vi "TLB Native Dynamic Events ver 0.26e.vi"() -> ()   [LabVIEW 2018] (continued)
          tunnel: w309 -> [_ _ _ _ _ _ _ _ _ _ _ _ _ _ _ _ _ _ _ _ _ _ _ _ _ _ _ _ _ _ _ _ _ _ _ _ _ _ _ _ _ _ _ _ _ _ _ _ _ _ _ _ _ _ _ _ _ _ _]
          tunnel: w308 -> [_ _ _ _ _ _ _ _ _ _ _ _ _ _ _ _ _ _ _ _ _ _ _ _ _ _ _ _ _ _ _ _ _ _ _ _ _ _ _ _ _ _ _ _ _ _ _ _ _ _ _ _ _ _ _ _ _ _ _]
          tunnel: w307 -> [_ _ _ _ _ _ _ _ _ _ _ _ _ _ _ _ _ _ _ _ _ _ _ _ _ _ _ _ _ _ _ _ _ _ _ _ _ _ _ _ _ _ _ _ _ _ _ _ _ _ _ _ _ _ _ _ _ _ _]
          tunnel: w306 -> [_ _ _ _ _ _ _ _ _ _ _ _ _ _ _ _ _ _ _ _ _ _ _ _ _ _ _ _ _ _ _ _ _ _ _ _ _ _ _ _ _ _ _ _ _ _ _ _ _ _ _ _ _ _ _ _ _ _ _]
          tunnel: w305 -> [_ _ _ _ _ _ _ _ _ _ _ _ _ _ _ _ _ _ _ _ _ _ _ _ _ _ _ _ _ _ _ _ _ _ _ _ _ _ _ _ _ _ _ _ _ _ _ _ _ _ _ _ _ _ _ _ _ _ _]
          tunnel: w304 -> [_ _ _ _ _ _ _ _ _ _ _ _ _ _ _ _ _ _ _ _ _ _ _ _ _ _ _ _ _ _ _ _ _ _ _ _ _ _ _ _ _ _ _ _ _ _ _ _ _ _ _ _ _ _ _ _ _ _ _]
          tunnel: w303 -> [_ _ _ _ _ _ _ _ _ _ _ _ _ _ _ _ _ _ _ _ _ _ _ _ _ _ _ _ _ _ _ _ _ _ _ _ _ _ _ _ _ _ w2205 _ w2299 _ _ _ _ _ _ _ _ _ _ w2816 _ _ _]
          tunnel: w302 -> [_ _ _ _ _ _ _ _ _ _ _ _ _ _ _ _ _ _ _ _ _ _ _ _ _ _ _ _ _ _ _ _ _ _ _ _ _ _ _ _ _ _ w2200 _ w2296 _ _ _ _ _ _ _ _ _ _ _ _ _ _]
          tunnel: [_ _ _ _ _ _ _ _ _ _ _ _ _ _ _ _ _ _ _ _ _ _ _ _ _ _ _ _ _ _ _ _ _ _ _ _ _ _ _ _ _ _ w2198 _ w2295 _ _ _ _ _ _ _ _ _ _ _ _ _ _] -> w301
          frame 0 {
            # ">>> yStepper command>>>"
          }
          frame 1 {
            # ">>> yStepper command>>>"
            n226 = for {
              shift-right: [w382] -> w376
              shift-left: w379 -> [w381]
              tunnel: string[] ["INIT", "RESET ARM", "RESET FLAGS", "RESET YAW", "NAVX CALIBRATE"] -> [w380] mode=indexing
              n227 = Enqueue Element(queue=w381, element=w380) -> (queue out=w382:refnum<queue>)  [unwired: 2 in, 2 out]
            }
            n228 = Bundle By Name(cluster=w374, "yStepper desired"=u8 0) -> (w373:T20)
            n229 = Bundle By Name(cluster=w371, "ySpeed"=0.0, "xSpeed"=0.0, "wSpeed"=0.0) -> (w370:T19)
          }
          frame 3 {
            # ">>Action Queue>>"
            # ">>> Motor control cluster >>>"
            # ">>> yStepper command>>>"
            n230 = Flush Queue(queue=w389, error in (no error)=w388) -> ()  [unwired: 3 out]
            n231 = for {
              shift-right: [w395] -> w390
              shift-left: w391 -> [w394]
              tunnel: string[] ["STOP", "RESET ENCODERS", "RESET YAW", "RESET ARM", "RESET ALL SENSORS", "DISPOSE CAM BUFFERS", "DISPOSE PROC BUFFERS", "CAM CLOSE", ""] -> [w393] mode=indexing
              n232 = Enqueue Element(queue=w394, element=w393) -> (queue out=w395:refnum<queue>)  [unwired: 2 in, 2 out]
            }
          }
          frame 4, Default {
            # ">>> Motor control cluster >>>"
            # ">>> yStepper command>>>"
            n233 = Dequeue Element(queue=w407, timeout in ms (-1)=w406, error in (no error)=w402) -> (element=w405:T10)  [unwired: 3 out]
            n234 = case shown="\"Start Task 9\"" w405 {
              tunnel: [w410 w418 w426 w434 w442 w450 w458 w466 w474 w481 w491 w499 w506 w509] -> w401
              tunnel: w404 -> [w411 w419 w427 w435 w443 w451 w459 w467 w475 w482 w490 w498 w506 w510]
              tunnel: [State_Type_Definitions,_for_0.26g_versions_and_later_2."Task 1A" ("Enum") State_Type_Definitions,_for_0.26g_versions_and_later_2."Task 2:Raise Arm" ("Enum") State_Type_Definitions,_for_0.26g_versions_and_later_2."Task 3" ("Enum") State_Type_Definitions,_for_0.26g_versions_and_later_2."Task 4_A" ("Enum") State_Type_Definitions,_for_0.26g_versions_and_later_2."Task 5A" ("Enum") State_Type_Definitions,_for_0.26g_versions_and_later_2."Task 6_A" ("Enum") State_Type_Definitions,_for_0.26g_versions_and_later_2."Task 8A: RAISE ARM" ("Enum") State_Type_Definitions,_for_0.26g_versions_and_later_2."Task 8A: RAISE ARM" ("Enum") State_Type_Definitions,_for_0.26g_versions_and_later_2."Task 8A: RAISE ARM" ("Enum") State_Type_Definitions,_for_0.26g_versions_and_later_2."Task 8A: RAISE ARM" ("Enum") State_Type_Definitions,_for_0.26g_versions_and_later_2."Task 9A: Raise Arm" ("Enum") State_Type_Definitions,_for_0.26g_versions_and_later_2."Task A1: Task 9 Open cam" ("Enum") State_Type_Definitions,_for_0.26g_versions_and_later_2."Idle" ("Enum") State_Type_Definitions,_for_0.26g_versions_and_later_2."Shutdown" ("Enum")] -> w403
              tunnel: [enum16{"Ball", "Soap", "Gel", "Pipe", "None"}."None" ("Object recognition mode") enum16{"Ball", "Soap", "Gel", "Pipe", "None"}."None" ("Object recognition mode") enum16{"Ball", "Soap", "Gel", "Pipe", "None"}."None" ("Object recognition mode") enum16{"Ball", "Soap", "Gel", "Pipe", "None"}."None" ("Object recognition mode") enum16{"Ball", "Soap", "Gel", "Pipe", "None"}."None" ("Object recognition mode") enum16{"Ball", "Soap", "Gel", "Pipe", "None"}."None" ("Object recognition mode") enum16{"Ball", "Soap", "Gel", "Pipe", "None"}."Ball" ("Object recognition mode") enum16{"Ball", "Soap", "Gel", "Pipe", "None"}."Gel" ("Object recognition mode") enum16{"Ball", "Soap", "Gel", "Pipe", "None"}."Pipe" ("Object recognition mode") enum16{"Ball", "Soap", "Gel", "Pipe", "None"}."Soap" ("Object recognition mode") enum16{"Ball", "Soap", "Gel", "Pipe", "None"}."None" ("Object recognition mode") enum16{"Ball", "Soap", "Gel", "Pipe", "None"}."None" ("Object recognition mode") enum16{"Ball", "Soap", "Gel", "Pipe", "None"}."None" ("Object recognition mode") enum16{"Ball", "Soap", "Gel", "Pipe", "None"}."None" ("Object recognition mode")] -> w396
              frame "Start Task 1" {
                n235 = for {
                  shift-right: [w415] -> w410
                  shift-left: w411 -> [w414]
                  tunnel: string[] ["RESET ENCODERS", "RESET YAW", "FORWARD", "READ ENCODERS"] -> [w413] mode=indexing
                  n236 = Enqueue Element(queue=w414, element=w413) -> (queue out=w415:refnum<queue>)  [unwired: 2 in, 2 out]
                }
              }
              frame "Start Task 2" {
                n237 = for {
                  shift-right: [w423] -> w418
                  shift-left: w419 -> [w422]
                  tunnel: string[] ["RESET ENCODERS", "RESET YAW", "READ ULTRASONIC", "ARDUINO - ULTRASONIC"] -> [w421] mode=indexing
                  n238 = Enqueue Element(queue=w422, element=w421) -> (queue out=w423:refnum<queue>)  [unwired: 2 in, 2 out]
                }
              }
              frame "Start Task 3" {
                n239 = for {
                  shift-right: [w431] -> w426
                  shift-left: w427 -> [w430]
                  tunnel: string[] ["RESET ENCODERS", "READ ENCODERS", "R-ACW"] -> [w429] mode=indexing
                  n240 = Enqueue Element(queue=w430, element=w429) -> (queue out=w431:refnum<queue>)  [unwired: 2 in, 2 out]
                }
              }
              frame "Start Task 4" {
                n241 = for {
                  shift-right: [w439] -> w434
                  shift-left: w435 -> [w438]
                  tunnel: string[] ["RESET YAW", "RESET ENCODERS", "RESET ARM", "RESET FLAGS", "", ""] -> [w437] mode=indexing
                  n242 = Enqueue Element(queue=w438, element=w437) -> (queue out=w439:refnum<queue>)  [unwired: 2 in, 2 out]
                }
              }
              frame "Start Task 5" {
                n243 = for {
                  shift-right: [w447] -> w442
                  shift-left: w443 -> [w446]
                  tunnel: string[] ["RESET YAW", "RESET ENCODERS", "RESET ARM", "RESET ALL SENSORS", "", ""] -> [w445] mode=indexing
                  n244 = Enqueue Element(queue=w446, element=w445) -> (queue out=w447:refnum<queue>)  [unwired: 2 in, 2 out]
                }
              }
              frame "Start Task 6" {
                n245 = for {
                  shift-right: [w455] -> w450
                  shift-left: w451 -> [w454]
                  tunnel: string[] ["OPEN LOG CAM ", "", "", "", "", ""] -> [w453] mode=indexing
                  n246 = Enqueue Element(queue=w454, element=w453) -> (queue out=w455:refnum<queue>)  [unwired: 2 in, 2 out]
                }
              }
              frame "Start Task 8 - BALL" {
                n247 = for {
                  shift-right: [w463] -> w458
                  shift-left: w459 -> [w462]
                  tunnel: string[] ["RESET YAW", "RESET ENCODERS", "RESET ARM", "RESET FLAGS"] -> [w461] mode=indexing
                  n248 = Enqueue Element(queue=w462, element=w461) -> (queue out=w463:refnum<queue>)  [unwired: 2 in, 2 out]
                }
              }
              frame "Start Task 8 - Gel" {
                n249 = for {
                  shift-right: [w471] -> w466
                  shift-left: w467 -> [w470]
                  tunnel: string[] ["RESET YAW", "RESET ENCODERS", "RESET ARM", "RESET FLAGS"] -> [w469] mode=indexing
                  n250 = Enqueue Element(queue=w470, element=w469) -> (queue out=w471:refnum<queue>)  [unwired: 2 in, 2 out]
                }
              }
              frame "Start Task 8 - Pipe" {
                n251 = for {
                  shift-right: [w479] -> w474
                  shift-left: w475 -> [w478]
                  tunnel: string[] ["RESET YAW", "RESET ENCODERS", "RESET ARM", "RESET FLAGS"] -> [w477] mode=indexing
                  n252 = Enqueue Element(queue=w478, element=w477) -> (queue out=w479:refnum<queue>)  [unwired: 2 in, 2 out]
                }
              }
              frame "Start Task 8 - Soap" {
                n253 = for {
                  shift-right: [w487] -> w481
                  shift-left: w482 -> [w486]
                  tunnel: string[] ["RESET YAW", "RESET ENCODERS", "RESET ARM", "RESET FLAGS"] -> [w485] mode=indexing
                  n254 = Enqueue Element(queue=w486, element=w485) -> (queue out=w487:refnum<queue>)  [unwired: 2 in, 2 out]
                }
              }
              frame "Start Task 9" {
                n255 = for {
                  shift-right: [w495] -> w491
                  shift-left: w490 -> [w494]
                  tunnel: string[] ["Z STEPPER BOX HEIGHT", "READ STEPPER VALUES", "", ""] -> [w493] mode=indexing
                  n256 = Enqueue Element(queue=w494, element=w493) -> (queue out=w495:refnum<queue>)  [unwired: 2 in, 2 out]
                }
              }
              frame "Start Task A" {
                n257 = for {
                  shift-right: [w503] -> w499
                  shift-left: w498 -> [w502]
                  tunnel: string[] ["RESET ENCODERS", "READ ENCODERS", "RESET YAW", "Z STEPPER BOX HEIGHT"] -> [w501] mode=indexing
                  n258 = Enqueue Element(queue=w502, element=w501) -> (queue out=w503:refnum<queue>)  [unwired: 2 in, 2 out]
                }
              }
              frame "None", Default {
              }
              frame "Exit" {
                n259 = for {
                  shift-right: [w514] -> w509
                  shift-left: w510 -> [w513]
                  tunnel: string[] ["STOP", "RESET ENCODERS", "RESET YAW", "EXIT"] -> [w512] mode=indexing
                  n260 = Enqueue Element(queue=w513, element=w512) -> (queue out=w514:refnum<queue>)  [unwired: 2 in, 2 out]
                }
              }
            }
          }
          frame 5 {
            # ">> Item Selection Bias >>"
            # ">>> yStepper command>>>"
            n261 = for {
              shift-right: [w525] -> w519
              shift-left: w521 -> [w524]
              tunnel: string[] ["INIT", "RESET ENCODERS", "RESET FLAGS", "CAM CLOSE", "DISPOSE BUFFERS", "EXIT", ""] -> [w523] mode=indexing
              n262 = Enqueue Element(queue=w524, element=w523) -> (queue out=w525:refnum<queue>)  [unwired: 2 in, 2 out]
            }
          }
          frame 6 {
            # ">>> Motor control cluster >>>"
            # ">> Line detection >>"
            # ">> Checks if 1 metre moved >>"
            # ">>> yStepper command>>>"
            # "Use 250"
            n263 = Greater?(x=w535, y=265.0) -> (0:w529:bool)
            n264 = Dequeue Element(queue=w542, timeout in ms (-1)=w541, error in (no error)=w540) -> (element=w539:T10)  [unwired: 3 out]
            n265 = And(x=w528, y=w529) -> (x .and. y?=w526:bool)
            n266 = case shown="\"Start Task 1\", Default" w539 {
              tunnel: w527 -> [w543 _]
              tunnel: [w553 State_Type_Definitions,_for_0.26g_versions_and_later_2."True Stop" ("Enum")] -> w538
              tunnel: w537 -> [w551 w568]
              tunnel: [w550 w567] -> w536
              tunnel: [State_Type_Definitions,_for_0.26g_versions_and_later_2."Idle" ("Enum") State_Type_Definitions,_for_0.26g_versions_and_later_2."Shutdown" ("Enum")] -> w533
              tunnel: w526 -> [w544 _]
              frame "Start Task 1", Default {
                n267 = Or(x=w544, y=w543) -> (x .or. y?=w545:bool)
                n268 = case shown="True" w545 {
                  tunnel: w551 -> [w556 w562]
                  tunnel: [w555 w560] -> w550
                  frame False {
                    n269 = for {
                      shift-right: [w558] -> w555
                      shift-left: w556 -> [w559]
                      tunnel: string[] ["READ ENCODERS", "READ NAVX", "FORWARD", "READ LINE SENSOR"] ("element") -> [w557] mode=indexing
                      n270 = Enqueue Element(queue=w559, element=w557) -> (queue out=w558:refnum<queue>)  [unwired: 2 in, 2 out]
                    }
                  }
                  frame True {
                    n271 = for {
                      shift-right: [w564] -> w560
                      shift-left: w562 -> [w565]
                      tunnel: string[] ["RESET YAW", "RESET ENCODERS", "STOP", ""] -> [w563] mode=indexing
                      n272 = Enqueue Element(queue=w565, element=w563) -> (queue out=w564:refnum<queue>)  [unwired: 2 in, 2 out]
                    }
                  }
                }
                n273 = Select(t=State_Type_Definitions,_for_0.26g_versions_and_later_2."True Stop" ("Enum"), s=w543, f=State_Type_Definitions,_for_0.26g_versions_and_later_2."Task 1B" ("Enum")) -> (s? t:f=w548:T18)
                n274 = Select(t=w548, s=w544, f=State_Type_Definitions,_for_0.26g_versions_and_later_2."Task 1A" ("Enum")) -> (s? t:f=w553:T18)
              }
              frame "Exit" {
                n275 = for {
                  shift-right: [w572] -> w567
                  shift-left: w568 -> [w573]
                  tunnel: string[] ["STOP", "RESET ENCODERS", "RESET YAW", ""] -> [w571] mode=indexing
                  n276 = Enqueue Element(queue=w573, element=w571) -> (queue out=w572:refnum<queue>)  [unwired: 2 in, 2 out]
                }
              }
            }
          }
          frame 7 {
            # ">>> Motor control cluster >>>"
            # ">> Line detection >>"
            # ">> Adds small distance overhead after 1M >>"
            # ">>> yStepper command>>>"
            n277 = Greater?(x=w580, y=50.0) -> (0:w574:bool)
            n278 = Dequeue Element(queue=w589, timeout in ms (-1)=w588, error in (no error)=w587) -> (element=w586:T10)  [unwired: 3 out]
            n279 = Or(x=w574, y=w581) -> (x .or. y?=w585:bool)
            n280 = case shown="\"Start Task 1\", Default" w586 {
              tunnel: w585 -> [w592 _]
              tunnel: [w596 State_Type_Definitions,_for_0.26g_versions_and_later_2."True Stop" ("Enum")] -> w584
              tunnel: w583 -> [w593 w611]
              tunnel: [w591 w610] -> w582
              tunnel: [State_Type_Definitions,_for_0.26g_versions_and_later_2."Idle" ("Enum") State_Type_Definitions,_for_0.26g_versions_and_later_2."Shutdown" ("Enum")] -> w578
              frame "Start Task 1", Default {
                n281 = case shown="True" w592 {
                  tunnel: w593 -> [w599 w605]
                  tunnel: [w598 w603] -> w591
                  frame False {
                    n282 = for {
                      shift-right: [w601] -> w598
                      shift-left: w599 -> [w602]
                      tunnel: string[] ["READ ENCODERS", "READ NAVX", "FORWARD", "READ LINE SENSOR"] ("element") -> [w600] mode=indexing
                      n283 = Enqueue Element(queue=w602, element=w600) -> (queue out=w601:refnum<queue>)  [unwired: 2 in, 2 out]
                    }
                  }
                  frame True {
                    n284 = for {
                      shift-right: [w607] -> w603
                      shift-left: w605 -> [w608]
                      tunnel: string[] ["RESET YAW", "RESET ENCODERS", "STOP", ""] -> [w606] mode=indexing
                      n285 = Enqueue Element(queue=w608, element=w606) -> (queue out=w607:refnum<queue>)  [unwired: 2 in, 2 out]
                    }
                  }
                }
                n286 = Select(t=State_Type_Definitions,_for_0.26g_versions_and_later_2."True Stop" ("Enum"), s=w592, f=State_Type_Definitions,_for_0.26g_versions_and_later_2."Task 1B" ("Enum")) -> (s? t:f=w596:T18)
              }
              frame "Exit" {
                n287 = for {
                  shift-right: [w615] -> w610
                  shift-left: w611 -> [w616]
                  tunnel: string[] ["STOP", "RESET ENCODERS", "RESET YAW", ""] -> [w614] mode=indexing
                  n288 = Enqueue Element(queue=w616, element=w614) -> (queue out=w615:refnum<queue>)  [unwired: 2 in, 2 out]
                }
              }
            }
          }
          frame 8 {
            # ">> Stepper height reeached >>"
            # ">>> yStepper command>>>"
            # ">> Manual override >>"
            n289 = Dequeue Element(queue=w622, timeout in ms (-1)=w621, error in (no error)=w620) -> (element=w631:T10)  [unwired: 3 out]
            n290 = Equal?(x=w624, y=u8 60) -> (x = y?=w629:bool)
            n291 = case shown="\"Start Task 1\", Default" w631 {
              tunnel: [w642 State_Type_Definitions,_for_0.26g_versions_and_later_2."True Stop" ("Enum")] -> w626
              tunnel: [w640 w657] -> w619
              tunnel: w628 -> [w639 _]
              tunnel: w627 -> [w633 _]
              tunnel: [State_Type_Definitions,_for_0.26g_versions_and_later_2."Idle" ("Enum") State_Type_Definitions,_for_0.26g_versions_and_later_2."Shutdown" ("Enum")] -> w625
              tunnel: w629 -> [w632 _]
              frame "Start Task 1", Default {
                # ">> WIill proceed to part ii if not manual override >>"
                # ">>If ENABLE or Trigger is set to true>>"
                n292 = Or(x=w632, y=w633) -> (x .or. y?=w634:bool)
                n293 = case shown="True" w632 {
                  tunnel: [w645 w651] -> w640
                  tunnel: w639 -> [w644 w650]
                  frame False {
                    n294 = for {
                      shift-right: [w647] -> w645
                      shift-left: w644 -> [w648]
                      tunnel: string[] ["Z STEPPER CAM HEIGHT", "READ STEPPER VALUES"] ("element") -> [w646] mode=indexing
                      n295 = Enqueue Element(queue=w648, element=w646) -> (queue out=w647:refnum<queue>)  [unwired: 2 in, 2 out]
                    }
                  }
                  frame True {
                    n296 = for {
                      shift-right: [w653] -> w651
                      shift-left: w650 -> [w654]
                      tunnel: string[] ["ARDUINO - ULTRASONIC", "READ ULTRASONIC", "", "", "", ""] -> [w652] mode=indexing
                      n297 = Enqueue Element(queue=w654, element=w652) -> (queue out=w653:refnum<queue>)  [unwired: 2 in, 2 out]
                    }
                  }
                }
                n298 = Select(t=State_Type_Definitions,_for_0.26g_versions_and_later_2."True Stop" ("Enum"), s=w633, f=State_Type_Definitions,_for_0.26g_versions_and_later_2."Task 2:Sensor Mode" ("Enum")) -> (s? t:f=w636:T18)
                n299 = Select(t=w636, s=w634, f=State_Type_Definitions,_for_0.26g_versions_and_later_2."Task 2:Raise Arm" ("Enum")) -> (s? t:f=w642:T18)
              }
              frame "Exit" {
                n300 = for {
                  shift-right: [w660] -> w657
                  shift-left: _ -> [w661]
                  tunnel: string[] ["STOP", "RESET ENCODERS", "RESET YAW", ""] -> [w659] mode=indexing
                  n301 = Enqueue Element(queue=w661, element=w659) -> (queue out=w660:refnum<queue>)  [unwired: 2 in, 2 out]
                }
              }
            }
          }
          frame 9 {
            w678 = u8 20 ("y")
            # ">>> yStepper command>>>"
            # ">>Object detected>>"
            n302 = Dequeue Element(queue=w671, timeout in ms (-1)=w670, error in (no error)=w669) -> (element=w679:T10)  [unwired: 3 out]
            n303 = Less?(x=w667, y=w678) -> (x < y?=w677:bool)
            n304 = Less?(x=w666, y=w678) -> (x < y?=w676:bool)
            n305 = Or(x=w677, y=w676) -> (x .or. y?=w662:bool)
            n306 = case shown="\"Start Task 1\", Default" w679 {
              tunnel: w662 -> [w682 _]
              tunnel: [w689 State_Type_Definitions,_for_0.26g_versions_and_later_2."True Stop" ("Enum")] -> w675
              tunnel: w668 -> [w681 _]
              tunnel: w672 -> [w688 w705]
              tunnel: [w687 w706] -> w674
              tunnel: [State_Type_Definitions,_for_0.26g_versions_and_later_2."Idle" ("Enum") State_Type_Definitions,_for_0.26g_versions_and_later_2."Shutdown" ("Enum")] -> w673
              frame "Start Task 1", Default {
                n307 = case shown="False" w682 {
                  tunnel: w688 -> [w692 w699]
                  tunnel: [w693 w698] -> w687
                  frame False {
                    n308 = for {
                      tunnel: string[] ["READ ULTRASONIC", "STOP"] ("element") -> [w694] mode=indexing
                      shift-right: [w696] -> w693
                      shift-left: w692 -> [w695]
                      n309 = Enqueue Element(queue=w695, element=w694) -> (queue out=w696:refnum<queue>)  [unwired: 2 in, 2 out]
                    }
                  }
                  frame True {
                    n310 = for {
                      shift-right: [w701] -> w698
                      shift-left: w699 -> [w702]
                      tunnel: string[] ["RESET ENCODERS", "READ NAVX", "READ ENCODERS"] -> [w700] mode=indexing
                      n311 = Enqueue Element(queue=w702, element=w700) -> (queue out=w701:refnum<queue>)  [unwired: 2 in, 2 out]
                    }
                  }
                }
                n312 = Or(x=w682, y=w681) -> (x .or. y?=w680:bool)
                n313 = Select(t=State_Type_Definitions,_for_0.26g_versions_and_later_2."True Stop" ("Enum"), s=w681, f=State_Type_Definitions,_for_0.26g_versions_and_later_2."Task 2:Reverse Mode" ("Enum")) -> (s? t:f=w683:T18)
                n314 = Select(t=w683, s=w680, f=State_Type_Definitions,_for_0.26g_versions_and_later_2."Task 2:Sensor Mode" ("Enum")) -> (s? t:f=w689:T18)
              }
              frame "Exit" {
                n315 = for {
                  shift-right: [w709] -> w706
                  shift-left: w705 -> [w710]
                  tunnel: string[] ["STOP", "RESET ENCODERS", "RESET YAW", "ARDUINO MODE 0"] -> [w708] mode=indexing
                  n316 = Enqueue Element(queue=w710, element=w708) -> (queue out=w709:refnum<queue>)  [unwired: 2 in, 2 out]
                }
              }
            }
          }
          frame 10 {
            # ">>> yStepper command>>>"
            n317 = Dequeue Element(queue=w721, timeout in ms (-1)=w722, error in (no error)=w723) -> (element=w725:T10)  [unwired: 3 out]
            n318 = Less?(x=w715, y=-50.0) -> (x < y?=w713:bool)
            n319 = case shown="\"Start Task 1\", Default" w725 {
              tunnel: [w735 State_Type_Definitions,_for_0.26g_versions_and_later_2."True Stop" ("Enum")] -> w717
              tunnel: w724 -> [w728 _]
              tunnel: w720 -> [w734 w751]
              tunnel: [w733 w752] -> w716
              tunnel: [State_Type_Definitions,_for_0.26g_versions_and_later_2."Idle" ("Enum") State_Type_Definitions,_for_0.26g_versions_and_later_2."Shutdown" ("Enum")] -> w718
              tunnel: w713 -> [w726 _]
              frame "Start Task 1", Default {
                n320 = case shown="True" w726 {
                  tunnel: w734 -> [w738 w745]
                  tunnel: [w739 w744] -> w733
                  frame False {
                    n321 = for {
                      tunnel: string[] ["READ ENCODERS", "REVERSE", "READ NAVX"] ("element") -> [w740] mode=indexing
                      shift-right: [w742] -> w739
                      shift-left: w738 -> [w741]
                      n322 = Enqueue Element(queue=w741, element=w740) -> (queue out=w742:refnum<queue>)  [unwired: 2 in, 2 out]
                    }
                  }
                  frame True {
                    n323 = for {
                      shift-right: [w747] -> w744
                      shift-left: w745 -> [w748]
                      tunnel: string[] ["STOP", "ARDUINO - ULTRASONIC", "READ ULTRASONIC", "RESET ENCODERS"] -> [w746] mode=indexing
                      n324 = Enqueue Element(queue=w748, element=w746) -> (queue out=w747:refnum<queue>)  [unwired: 2 in, 2 out]
                    }
                  }
                }
                n325 = Or(x=w726, y=w728) -> (x .or. y?=w727:bool)
                n326 = Select(t=State_Type_Definitions,_for_0.26g_versions_and_later_2."True Stop" ("Enum"), s=w728, f=State_Type_Definitions,_for_0.26g_versions_and_later_2."Task 2:Sensor Mode" ("Enum")) -> (s? t:f=w729:T18)
                n327 = Select(t=w729, s=w727, f=State_Type_Definitions,_for_0.26g_versions_and_later_2."Task 2:Reverse Mode" ("Enum")) -> (s? t:f=w735:T18)
              }
              frame "Exit" {
                n328 = for {
                  shift-right: [w755] -> w752
                  shift-left: w751 -> [w756]
                  tunnel: string[] ["STOP", "RESET ENCODERS", "RESET YAW", "ARDUINO MODE 0"] -> [w754] mode=indexing
                  n329 = Enqueue Element(queue=w756, element=w754) -> (queue out=w755:refnum<queue>)  [unwired: 2 in, 2 out]
                }
              }
            }
          }
          frame 11 {
            # ">>> Motor control cluster >>>"
            # ">>> yStepper command>>>"
            n330 = Dequeue Element(queue=w772, timeout in ms (-1)=w771, error in (no error)=w770) -> (element=w761:T10)  [unwired: 3 out]
            n331 = Less?(x=w769, y=-160.0) -> (x < y?=w766:bool)
            n332 = Or(x=w766, y=w767) -> (x .or. y?=w762:bool)
            n333 = case shown="\"Start Task 1\", Default" w761 {
              tunnel: w762 -> [w775 _]
              tunnel: [w779 State_Type_Definitions,_for_0.26g_versions_and_later_2."True Stop" ("Enum")] -> w763
              tunnel: w765 -> [w776 w795]
              tunnel: [w774 w794] -> w764
              tunnel: [State_Type_Definitions,_for_0.26g_versions_and_later_2."Idle" ("Enum") State_Type_Definitions,_for_0.26g_versions_and_later_2."Shutdown" ("Enum")] -> w760
              frame "Start Task 1", Default {
                n334 = case shown="False" w775 {
                  tunnel: w776 -> [w782 w788]
                  tunnel: [w781 w786] -> w774
                  frame False {
                    n335 = for {
                      shift-right: [w784] -> w781
                      shift-left: w782 -> [w785]
                      tunnel: string[] ["READ ENCODERS", "R-CW"] ("element") -> [w783] mode=indexing
                      n336 = Enqueue Element(queue=w785, element=w783) -> (queue out=w784:refnum<queue>)  [unwired: 2 in, 2 out]
                    }
                  }
                  frame True {
                    n337 = for {
                      shift-right: [w790] -> w786
                      shift-left: w788 -> [w791]
                      tunnel: string[] ["RESET YAW", "RESET ENCODERS", "STOP", "ARDUINO MODE 0"] -> [w789] mode=indexing
                      n338 = Enqueue Element(queue=w791, element=w789) -> (queue out=w790:refnum<queue>)  [unwired: 2 in, 2 out]
                    }
                  }
                }
                n339 = Select(t=State_Type_Definitions,_for_0.26g_versions_and_later_2."True Stop" ("Enum"), s=w775, f=State_Type_Definitions,_for_0.26g_versions_and_later_2."Task 3" ("Enum")) -> (s? t:f=w779:T18)
              }
              frame "Exit" {
                n340 = for {
                  shift-right: [w798] -> w794
                  shift-left: w795 -> [w799]
                  tunnel: string[] ["STOP", "RESET ENCODERS", "RESET YAW", ""] -> [w797] mode=indexing
                  n341 = Enqueue Element(queue=w799, element=w797) -> (queue out=w798:refnum<queue>)  [unwired: 2 in, 2 out]
                }
              }
            }
          }
          frame 12 {
            # ">> Stepper height reeached >>"
            # ">>> yStepper command>>>"
            # ">> Manual override >>"
            n342 = Dequeue Element(queue=w813, timeout in ms (-1)=w812, error in (no error)=w811) -> (element=w810:T10)  [unwired: 3 out]
            n343 = Equal?(x=w804, y=u8 60) -> (x = y?=w802:bool)
            n344 = case shown="\"Start Task 1\", Default" w810 {
              tunnel: [w825 State_Type_Definitions,_for_0.26g_versions_and_later_2."True Stop" ("Enum")] -> w809
              tunnel: [w823 w841] -> w808
              tunnel: w814 -> [w822 w838]
              tunnel: w807 -> [w816 _]
              tunnel: [State_Type_Definitions,_for_0.26g_versions_and_later_2."Idle" ("Enum") State_Type_Definitions,_for_0.26g_versions_and_later_2."Shutdown" ("Enum")] -> w806
              tunnel: w802 -> [w815 _]
              frame "Start Task 1", Default {
                # ">> WIill proceed to part ii if not manual override >>"
                # ">>If ENABLE or Trigger is set to true>>"
                n345 = Or(x=w815, y=w816) -> (x .or. y?=w817:bool)
                n346 = case shown="False" w815 {
                  tunnel: [w828 w834] -> w823
                  tunnel: w822 -> [w827 w833]
                  frame False {
                    n347 = for {
                      shift-right: [w830] -> w828
                      shift-left: w827 -> [w831]
                      tunnel: string[] ["Z STEPPER CAM HEIGHT", "READ STEPPER VALUES"] ("element") -> [w829] mode=indexing
                      n348 = Enqueue Element(queue=w831, element=w829) -> (queue out=w830:refnum<queue>)  [unwired: 2 in, 2 out]
                    }
                  }
                  frame True {
                    n349 = for {
                      shift-right: [w836] -> w834
                      shift-left: w833 -> [w837]
                      tunnel: string[] ["ARDUINO - ULTRASONIC", "READ ULTRASONIC", "FORWARD", "", "", ""] -> [w835] mode=indexing
                      n350 = Enqueue Element(queue=w837, element=w835) -> (queue out=w836:refnum<queue>)  [unwired: 2 in, 2 out]
                    }
                  }
                }
                n351 = Select(t=State_Type_Definitions,_for_0.26g_versions_and_later_2."True Stop" ("Enum"), s=w816, f=State_Type_Definitions,_for_0.26g_versions_and_later_2."Task 4_B" ("Enum")) -> (s? t:f=w819:T18)
                n352 = Select(t=w819, s=w817, f=State_Type_Definitions,_for_0.26g_versions_and_later_2."Task 4_A" ("Enum")) -> (s? t:f=w825:T18)
              }
              frame "Exit" {
                n353 = for {
                  shift-right: [w844] -> w841
                  shift-left: w838 -> [w845]
                  tunnel: string[] ["STOP", "RESET ENCODERS", "RESET YAW", ""] -> [w843] mode=indexing
                  n354 = Enqueue Element(queue=w845, element=w843) -> (queue out=w844:refnum<queue>)  [unwired: 2 in, 2 out]
                }
              }
            }
          }
          frame 13 {
            w851 = u8 20
            # ">> Path blocked >>"
            # ">>> yStepper command>>>"
            # ">> Manual override >>"
            n355 = Dequeue Element(queue=w860, timeout in ms (-1)=w859, error in (no error)=w858) -> (element=w857:T10)  [unwired: 3 out]
            n356 = Less?(x=w853, y=w851) -> (x < y?=w848:bool)
            n357 = Less?(x=w852, y=w851) -> (x < y?=w849:bool)
            n358 = And(x=w849, y=w848) -> (x .and. y?=w850:bool)
            n359 = case shown="\"Start Task 1\", Default" w857 {
              tunnel: [w874 State_Type_Definitions,_for_0.26g_versions_and_later_2."True Stop" ("Enum")] -> w862
              tunnel: [w872 w889] -> w863
              tunnel: w856 -> [w871 _]
              tunnel: w861 -> [w865 _]
              tunnel: [State_Type_Definitions,_for_0.26g_versions_and_later_2."Idle" ("Enum") State_Type_Definitions,_for_0.26g_versions_and_later_2."Shutdown" ("Enum")] -> w855
              tunnel: w850 -> [w864 _]
              frame "Start Task 1", Default {
                # ">> Manual override forces program to true stop >>"
                # ">>If ENABLE or Trigger is set to true>>"
                n360 = Or(x=w864, y=w865) -> (x .or. y?=w870:bool)
                n361 = case shown="False" w864 {
                  tunnel: [w877 w882] -> w872
                  tunnel: w871 -> [w876 w881]
                  frame False {
                    n362 = for {
                      shift-right: [w879] -> w877
                      shift-left: w876 -> [w880]
                      tunnel: string[] ["FORWARD", "READ ULTRASONIC", "READ NAVX"] ("element") -> [w878] mode=indexing
                      n363 = Enqueue Element(queue=w880, element=w878) -> (queue out=w879:refnum<queue>)  [unwired: 2 in, 2 out]
                    }
                  }
                  frame True {
                    n364 = for {
                      shift-right: [w885] -> w882
                      shift-left: w881 -> [w886]
                      tunnel: string[] ["STOP", "RESET YAW", "RESET ENCODERS", "RESET FLAGS"] -> [w884] mode=indexing
                      n365 = Enqueue Element(queue=w886, element=w884) -> (queue out=w885:refnum<queue>)  [unwired: 2 in, 2 out]
                    }
                  }
                }
                n366 = Select(t=State_Type_Definitions,_for_0.26g_versions_and_later_2."True Stop" ("Enum"), s=w865, f=State_Type_Definitions,_for_0.26g_versions_and_later_2."Task 4_C" ("Enum")) -> (s? t:f=w867:T18)
                n367 = Select(t=w867, s=w870, f=State_Type_Definitions,_for_0.26g_versions_and_later_2."Task 4_B" ("Enum")) -> (s? t:f=w874:T18)
              }
              frame "Exit" {
                n368 = for {
                  shift-right: [w892] -> w889
                  shift-left: _ -> [w893]
                  tunnel: string[] ["STOP", "RESET ENCODERS", "RESET YAW", ""] -> [w891] mode=indexing
                  n369 = Enqueue Element(queue=w893, element=w891) -> (queue out=w892:refnum<queue>)  [unwired: 2 in, 2 out]
                }
              }
            }
          }
          frame 14 {
            w905 = u8 20
            # ">> xDistance travelled>>"
            # ">> Path NOT blocked >>"
            # ">>> yStepper command>>>"
            # ">> Manual override >>"
            n370 = Dequeue Element(queue=w915, timeout in ms (-1)=w908, error in (no error)=w907) -> (element=w909:T10)  [unwired: 3 out]
            n371 = Greater?(x=w897, y=w905) -> (0:w903:bool)
            n372 = Greater?(x=w902, y=80.0) -> (0:w900:bool)
            n373 = Greater?(x=w896, y=w905) -> (0:w904:bool)
            n374 = And(x=w904, y=w903) -> (x .and. y?=w899:bool)
            n375 = And(x=w900, y=w899) -> (x .and. y?=w898:bool)
            n376 = case shown="\"Start Task 1\", Default" w909 {
              tunnel: [w926 State_Type_Definitions,_for_0.26g_versions_and_later_2."True Stop" ("Enum")] -> w912
              tunnel: [w924 w942] -> w911
              tunnel: w914 -> [w923 w939]
              tunnel: w913 -> [w917 _]
              tunnel: [State_Type_Definitions,_for_0.26g_versions_and_later_2."Idle" ("t") State_Type_Definitions,_for_0.26g_versions_and_later_2."Shutdown" ("Enum")] -> w910
              tunnel: w898 -> [w916 _]
              frame "Start Task 1", Default {
                # ">> Manual override forces program to true stop >>"
                # ">>If ENABLE or Trigger is set to true>>"
                n377 = Or(x=w916, y=w917) -> (x .or. y?=w922:bool)
                n378 = case shown="False" w916 {
                  tunnel: [w929 w934] -> w924
                  tunnel: w923 -> [w927 w933]
                  frame False {
                    n379 = for {
                      shift-right: [w931] -> w929
                      shift-left: w927 -> [w932]
                      tunnel: string[] ["RIGHT", "READ NAVX", "READ ENCODERS", "READ ULTRASONIC"] ("element") -> [w930] mode=indexing
                      n380 = Enqueue Element(queue=w932, element=w930) -> (queue out=w931:refnum<queue>)  [unwired: 2 in, 2 out]
                    }
                  }
                  frame True {
                    n381 = for {
                      shift-right: [w937] -> w934
                      shift-left: w933 -> [w938]
                      tunnel: string[] ["STOP", "RESET YAW", "RESET ENCODERS", "ARDUINO - ULTRASONIC"] -> [w936] mode=indexing
                      n382 = Enqueue Element(queue=w938, element=w936) -> (queue out=w937:refnum<queue>)  [unwired: 2 in, 2 out]
                    }
                  }
                }
                n383 = Select(t=State_Type_Definitions,_for_0.26g_versions_and_later_2."True Stop" ("Enum"), s=w917, f=State_Type_Definitions,_for_0.26g_versions_and_later_2."Task 4_D" ("Enum")) -> (s? t:f=w918:T18)
                n384 = Select(t=w918, s=w922, f=State_Type_Definitions,_for_0.26g_versions_and_later_2."Task 4_C" ("Enum")) -> (s? t:f=w926:T18)
              }
              frame "Exit" {
                n385 = for {
                  shift-right: [w945] -> w942
                  shift-left: w939 -> [w946]
                  tunnel: string[] ["STOP", "RESET ENCODERS", "RESET YAW", ""] -> [w944] mode=indexing
                  n386 = Enqueue Element(queue=w946, element=w944) -> (queue out=w945:refnum<queue>)  [unwired: 2 in, 2 out]
                }
              }
            }
          }
          frame 15 {
            w969 = u8 20
            # ">>> Motor control cluster >>>"
            # ">> Line detected >>"
            # ">> yDistance travelled>>"
            # ">> Path blocked >>"
            # ">>> yStepper command>>>"
            # ">> Manual override >>"
            n387 = Less?(x=w954, y=w969) -> (x < y?=w967:bool)
            n388 = Greater?(x=w958, y=200.0) -> (0:w965:bool)
            n389 = Less?(x=w953, y=w969) -> (x < y?=w968:bool)
            n390 = And(x=w968, y=w967) -> (x .and. y?=w964:bool)
            n391 = Dequeue Element(queue=w961, timeout in ms (-1)=w960, error in (no error)=w959) -> (element=w970:T10)  [unwired: 3 out]
            n392 = Or(x=w965, y=w964) -> (x .or. y?=w948:bool)
            n393 = And(x=w949, y=w948) -> (x .and. y?=w947:bool)
            n394 = case shown="\"Start Task 1\", Default" w970 {
              tunnel: [w981 State_Type_Definitions,_for_0.26g_versions_and_later_2."True Stop" ("Enum")] -> w957
              tunnel: [w979 w997] -> w955
              tunnel: w962 -> [w978 w994]
              tunnel: w963 -> [w972 _]
              tunnel: [State_Type_Definitions,_for_0.26g_versions_and_later_2."Idle" ("t") State_Type_Definitions,_for_0.26g_versions_and_later_2."Shutdown" ("Enum")] -> w956
              tunnel: w947 -> [w971 _]
              frame "Start Task 1", Default {
                # ">> Manual override forces program to true stop >>"
                # ">>If ENABLE or Trigger is set to true>>"
                n395 = Or(x=w971, y=w972) -> (x .or. y?=w977:bool)
                n396 = case shown="False" w971 {
                  tunnel: [w984 w989] -> w979
                  tunnel: w978 -> [w982 w988]
                  frame False {
                    n397 = for {
                      shift-right: [w986] -> w984
                      shift-left: w982 -> [w987]
                      tunnel: string[] ["FORWARD", "READ NAVX", "READ ENCODERS", "READ ULTRASONIC", "READ LINE SENSOR"] ("element") -> [w985] mode=indexing
                      n398 = Enqueue Element(queue=w987, element=w985) -> (queue out=w986:refnum<queue>)  [unwired: 2 in, 2 out]
                    }
                  }
                  frame True {
                    n399 = for {
                      shift-right: [w992] -> w989
                      shift-left: w988 -> [w993]
                      tunnel: string[] ["STOP", "RESET YAW", "RESET ENCODERS", "RESET FLAGS"] -> [w991] mode=indexing
                      n400 = Enqueue Element(queue=w993, element=w991) -> (queue out=w992:refnum<queue>)  [unwired: 2 in, 2 out]
                    }
                  }
                }
                n401 = Select(t=State_Type_Definitions,_for_0.26g_versions_and_later_2."True Stop" ("Enum"), s=w972, f=State_Type_Definitions,_for_0.26g_versions_and_later_2."True Stop" ("Enum")) -> (s? t:f=w973:T18)
                n402 = Select(t=w973, s=w977, f=State_Type_Definitions,_for_0.26g_versions_and_later_2."Task 4_D" ("Enum")) -> (s? t:f=w981:T18)
              }
              frame "Exit" {
                n403 = for {
                  shift-right: [w1000] -> w997
                  shift-left: w994 -> [w1001]
                  tunnel: string[] ["STOP", "RESET ENCODERS", "RESET YAW", ""] -> [w999] mode=indexing
                  n404 = Enqueue Element(queue=w1001, element=w999) -> (queue out=w1000:refnum<queue>)  [unwired: 2 in, 2 out]
                }
              }
            }
          }
          frame 16 {
            # "Stays in Task 5_A until stepper reaches desired \nheight"
            # ">>> Motor control cluster >>>"
            # ">>> yStepper command>>>"
            # ">> Manual override >>"
            n405 = Dequeue Element(queue=w1012, timeout in ms (-1)=w1011, error in (no error)=w1013) -> (element=w1010:T10)  [unwired: 3 out]
            n406 = Equal?(x=w1009, y=u8 1) -> (x = y?=w1007:bool)
            n407 = case shown="\"Start Task 1\", Default" w1010 {
              tunnel: [w1023 State_Type_Definitions,_for_0.26g_versions_and_later_2."True Stop" ("Enum")] -> w1014
              tunnel: [w1026 w1043] -> w1015
              tunnel: [State_Type_Definitions,_for_0.26g_versions_and_later_2."Idle" ("Enum") State_Type_Definitions,_for_0.26g_versions_and_later_2."Shutdown" ("Enum")] -> w1016
              tunnel: w1007 -> [w1022 _]
              tunnel: w1006 -> [w1021 _]
              tunnel: w1005 -> [w1017 w1040]
              frame "Start Task 1", Default {
                # "T: Go back to idle, F: Continue with task\""
                # ">> Manual override >>"
                n408 = case shown="True" w1022 {
                  tunnel: [w1030 w1036] -> w1026
                  tunnel: w1017 -> [w1028 w1034]
                  frame False {
                    n409 = for {
                      tunnel: string[] ["Z STEPPER GRAB HEIGHT", "READ STEPPER VALUES"] ("element") -> [w1031] mode=indexing
                      shift-right: [w1033] -> w1030
                      shift-left: w1028 -> [w1032]
                      n410 = Enqueue Element(queue=w1032, element=w1031) -> (queue out=w1033:refnum<queue>)  [unwired: 2 in, 2 out]
                    }
                  }
                  frame True {
                    n411 = for {
                      shift-right: [w1038] -> w1036
                      shift-left: w1034 -> [w1039]
                      tunnel: string[] ["SET TIMER 2", "", ""] -> [w1037] mode=indexing
                      n412 = Enqueue Element(queue=w1039, element=w1037) -> (queue out=w1038:refnum<queue>)  [unwired: 2 in, 2 out]
                    }
                  }
                }
                n413 = Or(x=w1022, y=w1021) -> (x .or. y?=w1024:bool)
                n414 = Select(t=State_Type_Definitions,_for_0.26g_versions_and_later_2."True Stop" ("Enum"), s=w1021, f=State_Type_Definitions,_for_0.26g_versions_and_later_2."Task 5B" ("Enum")) -> (s? t:f=w1018:T18)
                n415 = Select(t=w1018, s=w1024, f=State_Type_Definitions,_for_0.26g_versions_and_later_2."Task 5A" ("Enum")) -> (s? t:f=w1023:T18)
              }
              frame "Exit" {
                n416 = for {
                  shift-right: [w1046] -> w1043
                  shift-left: w1040 -> [w1047]
                  tunnel: string[] ["STOP", "RESET ENCODERS", "RESET YAW", "ARDUINO MODE 0"] -> [w1045] mode=indexing
                  n417 = Enqueue Element(queue=w1047, element=w1045) -> (queue out=w1046:refnum<queue>)  [unwired: 2 in, 2 out]
                }
              }
            }
          }
          frame 17 {
            # ">>> yStepper command>>>"
            n418 = Dequeue Element(queue=w1054, timeout in ms (-1)=w1053, error in (no error)=w1055) -> (element=w1052:T10)  [unwired: 3 out]
            n419 = case shown="\"Start Task 1\", Default" w1052 {
              tunnel: [w1067 State_Type_Definitions,_for_0.26g_versions_and_later_2."True Stop" ("Enum")] -> w1057
              tunnel: [w1070 w1087] -> w1056
              tunnel: [State_Type_Definitions,_for_0.26g_versions_and_later_2."Idle" ("Enum") State_Type_Definitions,_for_0.26g_versions_and_later_2."Shutdown" ("Enum")] -> w1058
              tunnel: w1060 -> [w1066 _]
              tunnel: w1059 -> [w1062 w1084]
              tunnel: w1048 -> [w1061 _]
              frame "Start Task 1", Default {
                # "T: Go back to idle, F: Continue with task\""
                # ">> Manual override >>"
                n420 = case shown="True" w1061 {
                  tunnel: [w1074 w1080] -> w1070
                  tunnel: w1062 -> [w1072 w1078]
                  frame False {
                    n421 = for {
                      tunnel: string[] ["CLOSE CLAW", "START TIMER", ""] ("element") -> [w1075] mode=indexing
                      shift-right: [w1077] -> w1074
                      shift-left: w1072 -> [w1076]
                      n422 = Enqueue Element(queue=w1076, element=w1075) -> (queue out=w1077:refnum<queue>)  [unwired: 2 in, 2 out]
                    }
                  }
                  frame True {
                    n423 = for {
                      shift-right: [w1082] -> w1080
                      shift-left: w1078 -> [w1083]
                      tunnel: string[] ["STOP", "", "", ""] -> [w1081] mode=indexing
                      n424 = Enqueue Element(queue=w1083, element=w1081) -> (queue out=w1082:refnum<queue>)  [unwired: 2 in, 2 out]
                    }
                  }
                }
                n425 = Or(x=w1061, y=w1066) -> (x .or. y?=w1068:bool)
                n426 = Select(t=State_Type_Definitions,_for_0.26g_versions_and_later_2."True Stop" ("Enum"), s=w1066, f=State_Type_Definitions,_for_0.26g_versions_and_later_2."Task 5C" ("Enum")) -> (s? t:f=w1063:T18)
                n427 = Select(t=w1063, s=w1068, f=State_Type_Definitions,_for_0.26g_versions_and_later_2."Task 5B" ("Enum")) -> (s? t:f=w1067:T18)
              }
              frame "Exit" {
                n428 = for {
                  shift-right: [w1090] -> w1087
                  shift-left: w1084 -> [w1091]
                  tunnel: string[] ["STOP", "RESET ENCODERS", "RESET YAW", "ARDUINO MODE 0"] -> [w1089] mode=indexing
                  n429 = Enqueue Element(queue=w1091, element=w1089) -> (queue out=w1090:refnum<queue>)  [unwired: 2 in, 2 out]
                }
              }
            }
          }
          frame 18 {
            # ">>> Motor control cluster >>>"
            # ">>> yStepper command>>>"
            # ">> Manual override >>"
            n430 = Equal?(x=w1094, y=u8 60) -> (x = y?=w1092:bool)
            n431 = Dequeue Element(queue=w1104, timeout in ms (-1)=w1103, error in (no error)=w1102) -> (element=w1101:T10)  [unwired: 3 out]
            n432 = case shown="\"Start Task 1\", Default" w1101 {
              tunnel: [w1113 State_Type_Definitions,_for_0.26g_versions_and_later_2."True Stop" ("Enum")] -> w1106
              tunnel: [w1116 w1133] -> w1099
              tunnel: [State_Type_Definitions,_for_0.26g_versions_and_later_2."Idle" ("Enum") State_Type_Definitions,_for_0.26g_versions_and_later_2."Shutdown" ("Enum")] -> w1098
              tunnel: w1100 -> [w1107 _]
              tunnel: w1105 -> [w1112 w1130]
              tunnel: w1092 -> [w1111 _]
              frame "Start Task 1", Default {
                # ">> Is time up? >>"
                # "Determines if object is in range to pick up"
                # ">> Manual override >>"
                n433 = case shown="True" w1111 {
                  tunnel: [w1120 w1126] -> w1116
                  tunnel: w1112 -> [w1118 w1124]
                  frame False {
                    n434 = for {
                      tunnel: string[] ["Z STEPPER CAM HEIGHT", "READ STEPPER VALUES"] ("element") -> [w1121] mode=indexing
                      shift-right: [w1123] -> w1120
                      shift-left: w1118 -> [w1122]
                      n435 = Enqueue Element(queue=w1122, element=w1121) -> (queue out=w1123:refnum<queue>)  [unwired: 2 in, 2 out]
                    }
                  }
                  frame True {
                    n436 = for {
                      shift-right: [w1128] -> w1126
                      shift-left: w1124 -> [w1129]
                      tunnel: string[] ["SET TIMER 5", "", ""] -> [w1127] mode=indexing
                      n437 = Enqueue Element(queue=w1129, element=w1127) -> (queue out=w1128:refnum<queue>)  [unwired: 2 in, 2 out]
                    }
                  }
                }
                n438 = Or(x=w1111, y=w1107) -> (x .or. y?=w1114:bool)
                n439 = Select(t=State_Type_Definitions,_for_0.26g_versions_and_later_2."True Stop" ("Enum"), s=w1107, f=State_Type_Definitions,_for_0.26g_versions_and_later_2."Task 5D" ("Enum")) -> (s? t:f=w1109:T18)
                n440 = Select(t=w1109, s=w1114, f=State_Type_Definitions,_for_0.26g_versions_and_later_2."Task 5C" ("Enum")) -> (s? t:f=w1113:T18)
              }
              frame "Exit" {
                n441 = for {
                  shift-right: [w1136] -> w1133
                  shift-left: w1130 -> [w1137]
                  tunnel: string[] ["STOP", "RESET ENCODERS", "RESET YAW", "ARDUINO MODE 0"] -> [w1135] mode=indexing
                  n442 = Enqueue Element(queue=w1137, element=w1135) -> (queue out=w1136:refnum<queue>)  [unwired: 2 in, 2 out]
                }
              }
            }
          }
          frame 19 {
            # ">>> yStepper command>>>"
            n443 = Dequeue Element(queue=w1145, timeout in ms (-1)=w1144, error in (no error)=w1143) -> (element=w1142:T10)  [unwired: 3 out]
            n444 = case shown="\"Start Task 1\", Default" w1142 {
              tunnel: [w1157 State_Type_Definitions,_for_0.26g_versions_and_later_2."True Stop" ("Enum")] -> w1149
              tunnel: [w1160 w1177] -> w1148
              tunnel: [State_Type_Definitions,_for_0.26g_versions_and_later_2."Idle" ("Enum") State_Type_Definitions,_for_0.26g_versions_and_later_2."Shutdown" ("Enum")] -> w1150
              tunnel: w1146 -> [w1156 _]
              tunnel: w1147 -> [w1152 w1174]
              tunnel: w1140 -> [w1151 _]
              frame "Start Task 1", Default {
                # ">> T: Breaks out of state loop; F: Stays in loop>>"
                # ">> Manual override >>"
                # ">> Checks if time is up>>"